vi "Dresden R2R Sputter 03.02.2018 IY24.vi"() -> ()   [LabVIEW 2009] (continued)
                n2407 = local read "RF 1 On"() -> (w4609:bool)
                n2408 = local read "Ch2_Tp_bv_on"() -> (w4633:bool)
                n2409 = local read "Ch2_pressure"() -> (w4594:dbl)
                n2410 = local read "Ch2_Mp_di"() -> (w4632:bool)
                n2411 = Less?(x=w4578, y=0.9) -> (x < y?=w4581:bool)
                n2412 = Less?(x=w4579, y=0.9) -> (x < y?=w4582:bool)
                n2413 = Less?(x=w4575, y=0.9) -> (x < y?=w4572:bool)
                n2414 = Less?(x=w4574, y=0.9) -> (x < y?=w4571:bool)
                n2415 = case shown="True" w4595 {
                  frame #0 {
                    n2416 = local read "Ch2_Pl_atm_di"() -> (w4649:bool)
                    n2417 = case shown="False" w4649 {
                      frame #0 {
                        n2418 = local write "Ch2_Tp_bv_open_safety"(TRUE ("Tp_bv_open_ch1_safety")) -> ()
                      }
                      frame #1 {
                        n2419 = local write "Ch2_Tp_bv_open_safety"(FALSE ("Tp_bv_open_ch1_safety")) -> ()
                      }
                    }
                  }
                  frame #1 {
                    n2420 = local read "Ch2_Pl_atm_di"() -> (w4652:bool)
                    n2421 = case shown="True" w4652 {
                      frame #0 {
                        n2422 = local write "Ch2_Tp_bv_open_safety"(FALSE ("Tp_bv_open_ch1_safety")) -> ()
                      }
                      frame #1 {
                        n2423 = local write "Ch2_Tp_bv_open_safety"(TRUE ("Tp_bv_open_ch1_safety")) -> ()
                      }
                    }
                  }
                }
                n2424 = Less?(x=w4563, y=0.9) -> (x < y?=w4560:bool)
                n2425 = Less?(x=w4562, y=0.9) -> (x < y?=w4559:bool)
                n2426 = Less?(x=w4625, y=0.01) -> (x < y?=w4622:bool)
                n2427 = local read "Ch2_Ds_di"() -> (w4587:bool)
                n2428 = Not(x=w4634) -> (.not. x?=w4635:bool)
                n2429 = Less?(x=w4598, y=0.1) -> (x < y?=w4602:bool)
                n2430 = Less?(x=w4554, y=0.08) -> (x < y?=w4597:bool)
                n2431 = Not(x=w4638) -> (.not. x?=w4637:bool)
                n2432 = Less?(x=w4556, y=0.08) -> (x < y?=w4619:bool)
                n2433 = Not(x=w4623) -> (.not. x?=w4613:bool)
                n2434 = Not And(1:w4601, 2:w4600) -> (0:w4603:bool)
                n2435 = Not(x=w4611) -> (.not. x?=w4610:bool)
                n2436 = Not(x=w4609) -> (.not. x?=w4608:bool)
                n2437 = Not(x=w4647) -> (.not. x?=w4643:bool)
                n2438 = Not(x=w4646) -> (.not. x?=w4644:bool)
                n2439 = Not(x=w4648) -> (.not. x?=w4645:bool)
                n2440 = Less Or Equal?(x=w4626, y=9e-05) -> (x <= y?=w4617:bool)
                n2441 = And(x=w4557, y=w4558) -> (x .and. y?=w4565:bool)
                n2442 = Not Or(1:w4628, 2:w4629) -> (0:w4630:bool)
                n2443 = Less?(x=w4555, y=0.08) -> (x < y?=w4606:bool)
                n2444 = And(x=w4581, y=w4582) -> (x .and. y?=w4584:bool)
                n2445 = Compound Arithmetic op=OR(w4641, w4640) -> (w4639:bool)
                n2446 = And(x=w4572, y=w4571) -> (x .and. y?=w4569:bool)
                n2447 = Less?(x=w4594, y=1.0) -> (x < y?=w4592:bool)
                n2448 = Not(x=w4591) -> (.not. x?=w4590:bool)
                n2449 = Compound Arithmetic op=AND(w4622, w4621, w4619) -> (w4618:bool)
                n2450 = And(x=w4560, y=w4559) -> (x .and. y?=w4566:bool)
                n2451 = And(x=w4602, y=w4603) -> (x .and. y?=w4604:bool)
                n2452 = local write "Ch2_Tp_bv_close_safety"(w4636) -> ()
                n2453 = Compound Arithmetic op=AND(w4645, w4644, w4643, w4607) -> (w4642:bool)
                n2454 = Not(x=w4639) -> (.not. x?=w4588:bool)
                n2455 = Compound Arithmetic op=AND(w4613, w4610, w4608) -> (w4612:bool)
                n2456 = Compound Arithmetic op=OR(w4633, w4632) -> (w4631:bool)
                n2457 = Or(x=w4583, y=w4584) -> (x .or. y?=w4585:bool)
                n2458 = Compound Arithmetic op=AND(w4617, w4616, w4615) -> (→"started_up_ch2":bool)
                n2459 = Or(x=w4570, y=w4569) -> (x .or. y?=w4568:bool)
                n2460 = Or(x=w4565, y=w4566) -> (x .or. y?=w4567:bool)
                n2461 = local write "Ch2_Cc_open_safety"(w4618) -> ()
                n2462 = local write "Ch2_Pl_vbv_open_safety"(w4630) -> ()
                n2463 = Compound Arithmetic op=AND(w4592, w4590) -> (w4589:bool)
                n2464 = local write "Ch2_sov_Ar_open_safety"(w4604) -> ()
                n2465 = local write "Ch2_WFC_close_safety"(w4612) -> ()
                n2466 = local write "Ch2_Ch_vbv_open_safety"(w4642) -> ()
                n2467 = local write "Ch2_sov_Ar_close_safety"(w4606) -> ()
                n2468 = local write "Ch2_Bg_bv_close_safety"(w4597) -> ()
                n2469 = local write "Ch2_Mp_stop_safety"(w4635) -> ()
                n2470 = And(x=w4588, y=w4587) -> (x .and. y?=w4586:bool)
                n2471 = local write "Ch2_Trns_gv_bp2_open_safety"(w4585) -> ()
                n2472 = local write "Ch2_Mp_stop_safety"(w4637) -> ()
                n2473 = local write "Ch2_Trns_gv_bp_open_safety"(w4568) -> ()
                n2474 = local write "Ch2_Bg_bv_open_safety"(w4589) -> ()
                n2475 = local write "Ch2_Tp_start_safety"(w4631) -> ()
                n2476 = local write "Ch2_Mp_start_safety"(w4586) -> ()
                n2477 = local write "Gv_open_ch2_3safety"(w4567) -> ()
              }
              frame #1 {
                w4655 = TRUE
                "Ch2_Bg_bv_open_safety" <- w4655
                "Ch2_Bg_bv_close_safety" <- w4655
                "Ch2_Tp_bv_open_safety" <- w4655
                "Ch2_Tp_bv_close_safety" <- w4655
                "Ch2_Ch_vbv_open_safety" <- w4655
                "Ch2_Ch_vbv_close_safety" <- w4655
                "Ch2_Bp_bv_open_R_safety" <- w4655
                "Ch2_Bp_bv_close_R_safety" <- w4655
                "Ch2_Bp_bv_open_L_safety" <- w4655
                "Ch2_Bp_bv_close_L_safety" <- w4655
                "Ch2_Trns_gv_bp2_open_safety" <- w4655
                "Ch2_Trns_gv_bp2_close_safety" <- w4655
                "Ch2_Trns_gv_bp_open_safety" <- w4655
                "Ch2_Trns_gv_bp_close_safety" <- w4655
                "Ch2_Cc_open_safety" <- w4655
                "Ch2_Cc_close_safety" <- w4655
                "Ch2_sov_Ar_open_safety" <- w4655
                "Ch2_sov_Ar_close_safety" <- w4655
                "Ch2_Mp_start_safety" <- w4655
                "Ch2_Mp_stop_safety" <- w4655
                "Ch2_Pl_vbv_open_safety" <- w4655
                "Ch2_Tp_start_safety" <- w4655
                "Ch2_Tp_stop_safety" <- w4655
                "Ch2_WFC_close_safety" <- w4655
                "Gv_close_ch2_3safety" <- w4655
                "Gv_open_ch2_3safety" <- w4655
              }
            }
            n2478 = case shown="False" "Security_cancel_ch4" {
              frame #0 {
                n2479 = local read "Ch4_Ch_atm_on"() -> (w4490:bool)
                n2480 = local read "Ar_sccm_act 4"() -> (w4485:dbl)
                n2481 = local read "Ch4pressure"() -> (w4538:dbl)
                n2482 = local read "Ar_sccm_act 4"() -> (w4483:dbl)
                n2483 = local read "Ch4pressure"() -> (w4539:dbl)
                n2484 = local read "Ch4_Tp_bv_on"() -> (w4528:bool)
                n2485 = local read "Ch4_Bg_bv_on"() -> (w4530:bool)
                n2486 = local read "Ch4_Ch_vbv_on"() -> (w4487:bool)
                n2487 = local read "TP4_working"() -> (w4523:bool)
                n2488 = local read "Ar_sccm_act 4"() -> (w4484:dbl)
                n2489 = local read "Dcps_is_on"() -> (w4513:bool)
                n2490 = local read "Ch4_Ch_cc_on"() -> (w4529:bool)
                n2491 = local read "Ch4_Tp_bv_on"() -> (w4525:bool)
                n2492 = local read "Ch4_Ch_vbv_on"() -> (w4499:bool)
                n2493 = local read "Tp4_stopped"() -> (w4507:bool)
                n2494 = local read "Ch4_Pc_bv_on"() -> (w4515:bool)
                n2495 = local read "Ch4_Ch_atm_on"() -> (w4498:bool)
                n2496 = local read "TP4_working"() -> (w4521:bool)
                n2497 = local read "Ch4_Pl_vbv_on"() -> (w4541:bool)
                n2498 = local read "RF 1 On"() -> (w4512:bool)
                n2499 = local read "Ch4_Ch_vbv_on"() -> (w4546:bool)
                n2500 = local read "Ch4_Tp_bv_on"() -> (w4544:bool)
                n2501 = local read "Ch4pressure"() -> (w4496:dbl)
                n2502 = local read "TP4_working"() -> (w4516:bool)
                n2503 = local read "Ch4_Mp_di"() -> (w4526:bool)
                n2504 = local read "Ch4pressure"() -> (w4505:dbl)
                n2505 = local read "Ch4_Tp_bv_on"() -> (w4534:bool)
                n2506 = local read "Tp4_stopped"() -> (w4542:bool)
                n2507 = local read "Ch4_Mp_di"() -> (w4535:bool)
                n2508 = case shown="True" w4490 {
                  frame #0 {
                    n2509 = local read "Ch4_Pl_atm_di"() -> (w4547:bool)
                    n2510 = case shown="False" w4547 {
                      frame #0 {
                        n2511 = local write "Ch4_Tp_bv_open_safety"(TRUE ("Tp_bv_open_ch1_safety")) -> ()
                      }
                      frame #1 {
                        n2512 = local write "Ch4_Tp_bv_open_safety"(FALSE ("Tp_bv_open_ch1_safety")) -> ()
                      }
                    }
                  }
                  frame #1 {
                    n2513 = local read "Ch4_Pl_atm_di"() -> (w4550:bool)
                    n2514 = case shown="False" w4550 {
                      frame #0 {
                        n2515 = local write "Ch4_Tp_bv_open_safety"(FALSE ("Tp_bv_open_ch1_safety")) -> ()
                      }
                      frame #1 {
                        n2516 = local write "Ch4_Tp_bv_open_safety"(TRUE ("Tp_bv_open_ch1_safety")) -> ()
                      }
                    }
                  }
                }
                n2517 = Less?(x=w4539, y=0.01) -> (x < y?=w4522:bool)
                n2518 = Less Or Equal?(x=w4538, y=9e-05) -> (x <= y?=w4517:bool)
                n2519 = Not(x=w4512) -> (.not. x?=w4509:bool)
                n2520 = Not(x=w4513) -> (.not. x?=w4510:bool)
                n2521 = Not(x=w4523) -> (.not. x?=w4511:bool)
                n2522 = Less?(x=w4483, y=0.08) -> (x < y?=w4503:bool)
                n2523 = local read "Ch4_Ds_di"() -> (w4492:bool)
                n2524 = Not(x=w4529) -> (.not. x?=w4524:bool)
                n2525 = Less?(x=w4485, y=0.08) -> (x < y?=w4519:bool)
                n2526 = Not(x=w4530) -> (.not. x?=w4532:bool)
                n2527 = Not(x=w4528) -> (.not. x?=w4531:bool)
                n2528 = Less?(x=w4496, y=0.1) -> (x < y?=w4500:bool)
                n2529 = Less?(x=w4484, y=0.08) -> (x < y?=w4495:bool)
                n2530 = Not And(1:w4499, 2:w4498) -> (0:w4501:bool)
                n2531 = Not(x=w4544) -> (.not. x?=w4543:bool)
                n2532 = Less?(x=w4505, y=1.0) -> (x < y?=w4488:bool)
                n2533 = Not Or(1:w4525, 2:w4526) -> (0:w4527:bool)
                n2534 = Not(x=w4487) -> (.not. x?=w4486:bool)
                n2535 = Compound Arithmetic op=OR(w4541, w4546) -> (w4545:bool)
                n2536 = Compound Arithmetic op=AND(w4531, w4532, w4524, w4507) -> (w4533:bool)
                n2537 = Compound Arithmetic op=AND(w4511, w4510, w4509) -> (w4508:bool)
                n2538 = Compound Arithmetic op=AND(w4517, w4516, w4515) -> (→"started_up_ch4":bool)
                n2539 = Compound Arithmetic op=AND(w4522, w4521, w4519) -> (w4518:bool)
                n2540 = Compound Arithmetic op=OR(w4534, w4535) -> (w4536:bool)
                n2541 = And(x=w4500, y=w4501) -> (x .and. y?=w4502:bool)
                n2542 = Not(x=w4545) -> (.not. x?=w4493:bool)
                n2543 = local write "Ch4_Tp_bv_close_safety"(w4542) -> ()
                n2544 = Compound Arithmetic op=AND(w4488, w4486) -> (w4489:bool)
                n2545 = local write "Ch4_Ch_vbv_open_safety"(w4533) -> ()
                n2546 = local write "Ch4_Pl_vbv_open_safety"(w4527) -> ()
                n2547 = local write "Ch4_Bg_bv_close_safety"(w4503) -> ()
                n2548 = local write "Ch4_WFC_close_safety"(w4508) -> ()
                n2549 = local write "Ch4_sov_Ar_close_safety"(w4495) -> ()
                n2550 = local write "Ch4_sov_Ar_open_safety"(w4502) -> ()
                n2551 = And(x=w4493, y=w4492) -> (x .and. y?=w4491:bool)
                n2552 = local write "Ch4_Bg_bv_open_safety"(w4489) -> ()
                n2553 = local write "Ch4_Mp_stop_safety"(w4543) -> ()
                n2554 = local write "Ch4_Cc_open_safety"(w4518) -> ()
                n2555 = local write "Ch4_Tp_start_safety"(w4536) -> ()
                n2556 = local write "Ch4_Mp_start_safety"(w4491) -> ()
              }
              frame #1 {
                w4553 = TRUE
                "Ch4_Bg_bv_open_safety" <- w4553
                "Ch4_Bg_bv_close_safety" <- w4553
                "Ch4_Tp_bv_open_safety" <- w4553
                "Ch4_Tp_bv_close_safety" <- w4553
                "Ch4_Ch_vbv_open_safety" <- w4553
                "Ch4_Ch_vbv_close_safety" <- w4553
                "Ch4_Bp_bv_open_L_safety" <- w4553
                "Ch4_Bp_bv_close_L_safety" <- w4553
                "Ch4_Trns_gv_bp_open_safety" <- w4553
                "Ch4_Trns_gv_bp_close_safety" <- w4553
                "Ch4_Cc_open_safety" <- w4553
                "Ch4_Cc_close_safety" <- w4553
                "Ch4_Mp_start_safety" <- w4553
                "Ch4_Mp_stop_safety" <- w4553
                "Ch4_Pl_vbv_open_safety" <- w4553
                "Ch4_Tp_start_safety" <- w4553
                "Ch4_Tp_stop_safety" <- w4553
                "Ch4_WFC_close_safety" <- w4553
                "Ch4_sov_Ar_open_safety" <- w4553
                "Ch4_sov_Ar_close_safety" <- w4553
              }
            }
            n2557 = case shown="False" "Security_cancel_ch3" {
              frame #0 {
                n2558 = local read "Ar_sccm_act 2"() -> (w4384:dbl)
                n2559 = local read "Ch3_pressure"() -> (w4475:dbl)
                n2560 = local read "Ch3_Ch_atm_on"() -> (w4423:bool)
                n2561 = local read "Ch3_Ch_vbv_on"() -> (w4457:bool)
                n2562 = local read "Ar_sccm_act 2"() -> (w4385:dbl)
                n2563 = local read "Ch3_Pl_vbv_on"() -> (w4458:bool)
                n2564 = local read "Ch3_Ds_di"() -> (w4421:bool)
                n2565 = local read "Ch3_Tp_bv_on"() -> (w4465:bool)
                n2566 = local read "Ch3_Bg_bv_on"() -> (w4463:bool)
                n2567 = local read "Ch3_Ch_cc_on"() -> (w4464:bool)
                n2568 = local read "Ch4_pressure2"() -> (w4395:dbl)
                n2569 = local read "Ch3_Ch_vbv_on"() -> (w4419:bool)
                n2570 = local read "Ch3_pressure2"() -> (w4394:dbl)
                n2571 = local read "Ch3_pressure2"() -> (w4398:dbl)
                n2572 = local read "Ch3_Tp_bv_on"() -> (w4468:bool)
                n2573 = local read "TP3_working"() -> (w4452:bool)
                n2574 = local read "Ch3_Ch_vbv_on"() -> (w4431:bool)
                n2575 = local read "Ch4_pressure2"() -> (w4399:dbl)
                n2576 = local read "Ch3_Tp_bv_on"() -> (w4424:bool)
                n2577 = local read "Ch3_pressure"() -> (w4472:dbl)
                n2578 = local read "TP3_working"() -> (w4455:bool)
                n2579 = local read "TP3_working"() -> (w4444:bool)
                n2580 = local read "TP3_working"() -> (w4443:bool)
                n2581 = local read "Tp3_stopped"() -> (w4445:bool)
                n2582 = local read "Ch3_Ch_atm_on"() -> (w4432:bool)
                n2583 = local read "Ch3_pressure2"() -> (w4409:dbl)
                n2584 = local read "Ch3_pressure"() -> (w4434:dbl)
                n2585 = local read "Ch4_pressure2"() -> (w4410:dbl)
                n2586 = local read "Ch3_Ch_atm_on"() -> (w4390:bool)
                n2587 = local read "Ch4_Ch_atm_on"() -> (w4414:bool)
                n2588 = local read "Ch3_Ch_atm_on"() -> (w4415:bool)
                n2589 = local read "Ch3_Tp_bv_on"() -> (w4471:bool)
                n2590 = local read "Ch3_Ch_atm_on"() -> (w4403:bool)
                n2591 = local read "Ch3_Pc_bv_on"() -> (w4447:bool)
                n2592 = local read "Ch3_Mp_di"() -> (w4467:bool)
                n2593 = local read "Ch3_pressure"() -> (w4437:dbl)
                n2594 = local read "Tp3_stopped"() -> (w4454:bool)
                n2595 = local read "TP3_working"() -> (w4448:bool)
                n2596 = local read "Ar_sccm_act 2"() -> (w4383:dbl)
                n2597 = local read "Ch3_Mp_di"() -> (w4470:bool)
                n2598 = Less?(x=w4475, y=0.01) -> (x < y?=w4453:bool)
                n2599 = Not(x=w4464) -> (.not. x?=w4460:bool)
                n2600 = Not(x=w4463) -> (.not. x?=w4461:bool)
                n2601 = Not(x=w4465) -> (.not. x?=w4462:bool)
                n2602 = Less?(x=w4385, y=0.08) -> (x < y?=w4451:bool)
                n2603 = Not(x=w4443) -> (.not. x?=w4440:bool)
                n2604 = Not(x=w4455) -> (.not. x?=w4442:bool)
                n2605 = Not(x=w4444) -> (.not. x?=w4441:bool)
                n2606 = Less?(x=w4395, y=0.9) -> (x < y?=w4392:bool)
                n2607 = Less?(x=w4394, y=0.9) -> (x < y?=w4391:bool)
                n2608 = Less?(x=w4398, y=0.9) -> (x < y?=w4401:bool)
                n2609 = Less?(x=w4399, y=0.9) -> (x < y?=w4402:bool)
                n2610 = Not(x=w4424) -> (.not. x?=w4425:bool)
                n2611 = Compound Arithmetic op=OR(w4458, w4457) -> (w4456:bool)
                n2612 = Less?(x=w4409, y=0.9) -> (x < y?=w4412:bool)
                n2613 = case shown="False" w4423 {
                  frame #0 {
                    n2614 = local read "Ch3_Pl_atm_di"() -> (w4476:bool)
                    n2615 = case shown="False" w4476 {
                      frame #0 {
                        n2616 = local write "Ch3_Tp_bv_open_safety"(TRUE ("Tp_bv_open_ch1_safety")) -> ()
                      }
                      frame #1 {
                        n2617 = local write "Ch3_Tp_bv_open_safety"(FALSE ("Tp_bv_open_ch1_safety")) -> ()
                      }
                    }
                  }
                  frame #1 {
                    n2618 = local read "Ch3_Pl_atm_di"() -> (w4479:bool)
                    n2619 = case shown="True" w4479 {
                      frame #0 {
                        n2620 = local write "Ch3_Tp_bv_open_safety"(FALSE ("Tp_bv_open_ch1_safety")) -> ()
                      }
                      frame #1 {
                        n2621 = local write "Ch3_Tp_bv_open_safety"(TRUE ("Tp_bv_open_ch1_safety")) -> ()
                      }
                    }
                  }
                }
                n2622 = Less?(x=w4434, y=0.1) -> (x < y?=w4430:bool)
                n2623 = Less?(x=w4384, y=0.08) -> (x < y?=w4435:bool)
                n2624 = Less?(x=w4410, y=0.9) -> (x < y?=w4413:bool)
                n2625 = Not And(1:w4431, 2:w4432) -> (0:w4429:bool)
                n2626 = Not Or(1:w4468, 2:w4467) -> (0:w4466:bool)
                n2627 = Less?(x=w4437, y=0.1) -> (x < y?=w4418:bool)
                n2628 = Not(x=w4419) -> (.not. x?=w4417:bool)
                n2629 = Less Or Equal?(x=w4472, y=9e-05) -> (x <= y?=w4449:bool)
                n2630 = Compound Arithmetic op=AND(w4462, w4461, w4460, w4445) -> (w4459:bool)
                n2631 = Less?(x=w4383, y=0.08) -> (x < y?=w4426:bool)
                n2632 = Not(x=w4456) -> (.not. x?=w4422:bool)
                n2633 = Compound Arithmetic op=OR(w4471, w4470) -> (w4469:bool)
                n2634 = Compound Arithmetic op=AND(w4442, w4441, w4440) -> (w4439:bool)
                n2635 = Compound Arithmetic op=AND(w4453, w4452, w4451) -> (w4450:bool)
                n2636 = And(x=w4430, y=w4429) -> (x .and. y?=w4428:bool)
                n2637 = And(x=w4415, y=w4414) -> (x .and. y?=w4407:bool)
                n2638 = local write "Ch3_Tp_bv_close_safety"(w4454) -> ()
                n2639 = And(x=w4392, y=w4391) -> (x .and. y?=w4389:bool)
                n2640 = And(x=w4422, y=w4421) -> (x .and. y?=w4420:bool)
                n2641 = And(x=w4401, y=w4402) -> (x .and. y?=w4404:bool)
                n2642 = local write "Ch3_Ch_vbv_open_safety"(w4459) -> ()
                n2643 = Compound Arithmetic op=AND(w4449, w4448, w4447) -> (→"started_up_ch3":bool)
                n2644 = And(x=w4412, y=w4413) -> (x .and. y?=w4387:bool)
                n2645 = local write "Ch3_Pl_vbv_open_safety"(w4466) -> ()
                n2646 = local write "Ch3_WFC_close_safety"(w4439) -> ()
                n2647 = local write "Ch3_sov_Ar_open_safety"(w4428) -> ()
                n2648 = Compound Arithmetic op=AND(w4418, w4417) -> (w4416:bool)
                n2649 = Or(x=w4390, y=w4389) -> (x .or. y?=w4388:bool)
                n2650 = Or(x=w4403, y=w4404) -> (x .or. y?=w4405:bool)
                n2651 = local write "Ch3_Mp_stop_safety"(w4425) -> ()
                n2652 = local write "Ch3_Bg_bv_close_safety"(w4435) -> ()
                n2653 = local write "Ch3_sov_Ar_close_safety"(w4426) -> ()
                n2654 = local write "Ch3_Cc_open_safety"(w4450) -> ()
                n2655 = Or(x=w4407, y=w4387) -> (x .or. y?=w4406:bool)
                n2656 = local write "Ch3_Tp_start_safety"(w4469) -> ()
                n2657 = local write "Ch3_Mp_start_safety"(w4420) -> ()
                n2658 = local write "Ch3_Trns_gv_bp2_open_safety"(w4388) -> ()
                n2659 = local write "Ch3_Trns_gv_bp_open_safety"(w4405) -> ()
                n2660 = local write "Ch3_Bg_bv_start_safety"(w4416) -> ()
                n2661 = local write "Gv_open_ch3_4safety"(w4406) -> ()
              }
              frame #1 {
                w4482 = TRUE
                "Ch3_Bg_bv_start_safety" <- w4482
                "Ch3_Bg_bv_close_safety" <- w4482
                "Ch3_Tp_bv_open_safety" <- w4482
                "Ch3_Tp_bv_close_safety" <- w4482
                "Ch3_Ch_vbv_open_safety" <- w4482
                "Ch3_Ch_vbv_close_safety" <- w4482
                "Ch3_Bp_bv_open_R_safety" <- w4482
                "Ch3_Bp_bv_close_R_safety" <- w4482
                "Ch3_Bp_bv_close_L_safety" <- w4482
                "Ch3_Bp_bv_open_L_safety" <- w4482
                "Ch3_Trns_gv_bp2_close_safety" <- w4482
                "Ch3_Trns_gv_bp2_open_safety" <- w4482
                "Ch3_Trns_gv_bp_open_safety" <- w4482
                "Ch3_Trns_gv_bp_close_safety" <- w4482
                "Ch3_Cc_open_safety" <- w4482
                "Ch3_Cc_close_safety" <- w4482
                "Ch3_sov_Ar_open_safety" <- w4482
                "Ch3_sov_Ar_close_safety" <- w4482
                "Ch3_Mp_start_safety" <- w4482
                "Ch3_Mp_stop_safety" <- w4482
                "Ch3_Pl_vbv_open_safety" <- w4482
                "Ch3_Tp_start_safety" <- w4482
                "Ch3_Tp_stop_safety" <- w4482
                "Ch3_WFC_close_safety" <- w4482
                "Gv_open_ch3_4safety" <- w4482
                "Gv_close_ch3_4safety" <- w4482
              }
            }
          }
        }
        n2662 = stacked-sequence {
          frame #0 {
            # "GAS FLOW CONTROL"
            n2663 = Or(x="Ar_set_zero_ch1", y="Ar_auto_set_zero_ch1") -> (x .or. y?=w4321:bool)
            n2664 = Or(x="Ar_set_zero_ch2", y="Ar_auto_set_zero_ch2") -> (x .or. y?=w4311:bool)
            n2665 = case shown="True" "Mfc_Ar _set 2" {
              frame #0 {
              }
              frame #1 {
                n2666 = stacked-sequence {
                  frame #0 {
                    n2667 = local write "Ar_sccm1_2"(u16 0 ("Ar_sccm 2")) -> ()
                  }
                  frame #1 {
                    n2668 = Wait (ms)(milliseconds to wait=u32 200) -> ()  [unwired: 1 out]
                  }
                  frame #2 {
                    n2669 = local write "Mfc_Ar _1_2_set"(TRUE ("Ar_set_ch1")) -> ()
                  }
                  frame #3 {
                    n2670 = Wait (ms)(milliseconds to wait=u32 1000) -> ()  [unwired: 1 out]
                  }
                  frame #4 {
                    n2671 = local write "Mfc_Ar _1_2_set"(FALSE ("Ar_set_ch1")) -> ()
                  }
                  frame #5 {
                    n2672 = Wait (ms)(milliseconds to wait=u32 200) -> ()  [unwired: 1 out]
                  }
                  frame #6 {
                    n2673 = local write "Ar_sccm1_2"("Ar_sccm 2") -> ()
                  }
                  frame #7 {
                    n2674 = Wait (ms)(milliseconds to wait=u32 200) -> ()  [unwired: 1 out]
                  }
                  frame #8 {
                    n2675 = local write "Mfc_Ar _1_2_set"(TRUE ("Ar_set_ch1")) -> ()
                  }
                  frame #9 {
                    n2676 = Wait (ms)(milliseconds to wait=u32 1000) -> ()  [unwired: 1 out]
                  }
                  frame #10 {
                    n2677 = local write "Mfc_Ar _set 2"(FALSE ("Mfc_Ar _set 2")) -> ()
                  }
                }
              }
            }
            n2678 = case shown="True" w4311 {
              frame #0 {
              }
              frame #1 {
                n2679 = flat-sequence {
                  frame #0 {
                    n2680 = local write "Ar_sccm1_2"(u16 0 ("Ar_sccm 2")) -> ()
                  }
                  frame #1 {
                    n2681 = Wait (ms)(milliseconds to wait=u32 200) -> ()  [unwired: 1 out]
                  }
                  frame #2 {
                    n2682 = local write "Ar_auto_set_zero_ch2"(FALSE ("Ar_auto_set_zero_ch2")) -> ()
                    n2683 = local write "Mfc_Ar _1_2_set"(TRUE ("Ar_set_ch1")) -> ()
                  }
                }
              }
            }
            n2684 = case shown="True" w4321 {
              frame #0 {
              }
              frame #1 {
                n2685 = flat-sequence {
                  frame #0 {
                    n2686 = local write "Ar_sccm1_2"(u16 0 ("Ar_sccm 2")) -> ()
                  }
                  frame #1 {
                    n2687 = Wait (ms)(milliseconds to wait=u32 200) -> ()  [unwired: 1 out]
                  }
                  frame #2 {
                    n2688 = local write "Ar_auto_set_zero_ch1"(FALSE ("Ar_auto_set_zero_ch1")) -> ()
                    n2689 = local write "Mfc_Ar _1_2_set"(TRUE ("Ar_set_ch1")) -> ()
                  }
                }
              }
            }
            n2690 = case shown="True" "Mfc2_Ar _set4" {
              frame #0 {
              }
              frame #1 {
                n2691 = stacked-sequence {
                  frame #0 {
                    n2692 = local write "Ar_sccm3_4"(u16 0 ("Ar_sccm3_4")) -> ()
                  }
                  frame #1 {
                    n2693 = Wait (ms)(milliseconds to wait=u32 200) -> ()  [unwired: 1 out]
                  }
                  frame #2 {
                    n2694 = local write "Mfc2_Ar _3_4_set"(TRUE ("Mfc2_Ar _set")) -> ()
                  }
                  frame #3 {
                    n2695 = Wait (ms)(milliseconds to wait=u32 1000) -> ()  [unwired: 1 out]
                  }
                  frame #4 {
                    n2696 = local write "Ar_sccm3_4"("Ar_sccm4") -> ()
                  }
                  frame #5 {
                    n2697 = Wait (ms)(milliseconds to wait=u32 200) -> ()  [unwired: 1 out]
                  }
                  frame #6 {
                    n2698 = local write "Mfc2_Ar _3_4_set"(TRUE ("Mfc2_Ar _set")) -> ()
                  }
                  frame #7 {
                    n2699 = Wait (ms)(milliseconds to wait=u32 1000) -> ()  [unwired: 1 out]
                  }
                  frame #8 {
                    n2700 = local write "Mfc2_Ar _set4"(FALSE ("Mfc2_Ar _set4")) -> ()
                  }
                }
              }
            }
            n2701 = case shown="True" "Mfc_Ar _set" {
              frame #0 {
              }
              frame #1 {
                n2702 = stacked-sequence {
                  frame #0 {
                    n2703 = local write "Ar_sccm1_2"(u16 0 ("Ar_sccm 2")) -> ()
                  }
                  frame #1 {
                    n2704 = Wait (ms)(milliseconds to wait=u32 200) -> ()  [unwired: 1 out]
                  }
                  frame #2 {
                    n2705 = local write "Mfc_Ar _1_2_set"(TRUE ("Ar_set_ch1")) -> ()
                  }
                  frame #3 {
                    n2706 = Wait (ms)(milliseconds to wait=u32 1000) -> ()  [unwired: 1 out]
                  }
                  frame #4 {
                    n2707 = local write "Mfc_Ar _1_2_set"(FALSE ("Ar_set_ch1")) -> ()
                  }
                  frame #5 {
                    n2708 = Wait (ms)(milliseconds to wait=u32 200) -> ()  [unwired: 1 out]
                  }
                  frame #6 {
                    n2709 = local write "Ar_sccm1_2"("Ar_sccm") -> ()
                  }
                  frame #7 {
                    n2710 = Wait (ms)(milliseconds to wait=u32 200) -> ()  [unwired: 1 out]
                  }
                  frame #8 {
                    n2711 = local write "Mfc_Ar _1_2_set"(TRUE ("Ar_set_ch1")) -> ()
                  }
                  frame #9 {
                    n2712 = Wait (ms)(milliseconds to wait=u32 1000) -> ()  [unwired: 1 out]
                  }
                  frame #10 {
                    n2713 = local write "Mfc_Ar _set"(FALSE ("Mfc_Ar _set")) -> ()
                  }
                }
              }
            }
            n2714 = case shown="True" "Mfc2_Ar _set3" {
              frame #0 {
              }
              frame #1 {
                n2715 = stacked-sequence {
                  frame #0 {
                    n2716 = local write "Ar_sccm3_4"(u16 0 ("Ar_sccm3_4")) -> ()
                  }
                  frame #1 {
                    n2717 = Wait (ms)(milliseconds to wait=u32 200) -> ()  [unwired: 1 out]
                  }
                  frame #2 {
                    n2718 = local write "Mfc2_Ar _3_4_set"(TRUE ("Mfc2_Ar _set")) -> ()
                  }
                  frame #3 {
                    n2719 = Wait (ms)(milliseconds to wait=u32 1000) -> ()  [unwired: 1 out]
                  }
                  frame #4 {
                    n2720 = local write "Ar_sccm3_4"("Ar_sccm3") -> ()
                  }
                  frame #5 {
                    n2721 = Wait (ms)(milliseconds to wait=u32 200) -> ()  [unwired: 1 out]
                  }
                  frame #6 {
                    n2722 = local write "Mfc2_Ar _3_4_set"(TRUE ("Mfc2_Ar _set")) -> ()
                  }
                  frame #7 {
                    n2723 = Wait (ms)(milliseconds to wait=u32 1000) -> ()  [unwired: 1 out]
                  }
                  frame #8 {
                    n2724 = local write "Mfc2_Ar _set3"(FALSE ("Mfc2_Ar _set3")) -> ()
                  }
                }
              }
            }
            n2725 = Or(x="Ar_set_zero_ch4", y="Ar_auto_set_zero_ch4") -> (x .or. y?=w4313:bool)
            n2726 = Or(x="Ar_set_zero_ch3", y="Ar_auto_set_zero_ch3") -> (x .or. y?=w4316:bool)
            n2727 = case shown="True" w4313 {
              frame #0 {
              }
              frame #1 {
                n2728 = flat-sequence {
                  frame #0 {
                    n2729 = local write "Ar_sccm3_4"(u16 0 ("Ar_sccm2 2")) -> ()
                  }
                  frame #1 {
                    n2730 = Wait (ms)(milliseconds to wait=u32 200) -> ()  [unwired: 1 out]
                  }
                  frame #2 {
                    n2731 = local write "Mfc2_Ar _3_4_set"(TRUE ("Mfc2_Ar _set")) -> ()
                    n2732 = local write "Ar_auto_set_zero_ch4"(FALSE ("Ar_auto_set_zero_ch4")) -> ()
                  }
                }
              }
            }
            n2733 = case shown="True" w4316 {
              frame #0 {
              }
              frame #1 {
                n2734 = flat-sequence {
                  frame #0 {
                    n2735 = local write "Ar_sccm3_4"(u16 0 ("Ar_sccm2 2")) -> ()
                  }
                  frame #1 {
                    n2736 = Wait (ms)(milliseconds to wait=u32 200) -> ()  [unwired: 1 out]
                  }
                  frame #2 {
                    n2737 = local write "Ar_auto_set_zero_ch3"(FALSE ("Ar_auto_set_zero_ch3")) -> ()
                    n2738 = local write "Mfc2_Ar _3_4_set"(TRUE ("Mfc2_Ar _set")) -> ()
                  }
                }
              }
            }
          }
        }
        n2739 = stacked-sequence {
          frame #0 {
            # "Process Flow"
            n2740 = case shown="True" "Ppsok" {
              frame #0 {
              }
              frame #1 {
                n2741 = stacked-sequence {
                  frame #0 {
                    n2742 = local read "Pps_code_entry"() -> (w5512:string)
                    n2743 = Equal?(x=w5512, y="PF227= ") -> (x = y?=w5510:bool)
                    n2744 = Read from Text File(file (use dialog)="Process_flow_messages") -> (text=w5520:string)  [unwired: 3 in, 3 out]
                    n2745 = Match Pattern(string=w5520, regular expression="Pps_code_entry") -> (after substring=w5521:string)  [unwired: 1 in, 3 out]
                    n2746 = case shown="False" w5510 {
                      tunnel: [w5522 "                "] -> w5509
                      frame #0 {
                        n2747 = Get Date/Time String() -> (date string=w5525:string, time string=w5523:string)  [unwired: 3 in]
                        n2748 = Concatenate Strings(w5525, " / " ("string"), w5523) -> (w5522:string)
                      }
                      frame #1 {
                      }
                    }
                    n2749 = Match Pattern(string=w5521, regular expression="***") -> (before substring=w5516:string)  [unwired: 1 in, 3 out]
                    n2750 = Concatenate Strings(w5509, w5516) -> (w5514:string)
                    n2751 = String Length(string=w5516) -> (length=w5517:i32)
                    n2752 = Not Equal To 0?(x=w5517) -> (x != 0?=w5515:bool)
                    n2753 = case shown="True" w5515 {
                      tunnel: w5514 -> [_ w5532]
                      frame #0 {
                      }
                      frame #1 {
                        n2754 = property on="Process_flow" class="Str"() -> ("Text.Scroll Position"=w5529:u32)  [unwired: 2 in, 2 out]
                        n2755 = local read "Process_flow"() -> (w5530:string)
                        n2756 = Concatenate Strings(w5530, "\r", w5532) -> (w5527:string)
                        n2757 = Add(x=w5529, y=u32 10) -> (x+y=w5528:u32)
                        n2758 = local write "Process_flow"(w5527) -> ()
                        n2759 = property on="Process_flow" class="Str"("Text.Scroll Position"=w5528) -> ()  [unwired: 2 in, 2 out]
                      }
                    }
                  }
                  frame #1 {
                    n2760 = Wait (ms)(milliseconds to wait=u32 100) -> ()  [unwired: 1 out]
                  }
                  frame #2 {
                    n2761 = local write "Ppsok"(FALSE ("PPSOK")) -> ()
                  }
                }
              }
            }
          }
        }
        n2762 = stacked-sequence {
          frame #0 {
            # "INSTANT MESSAGES"
            n2763 = local read "Ch3_Ch_vbv_on"() -> (w4843:bool)
            n2764 = local read "Ch3_Bp_bv_on_L"() -> (w4908:bool)
            n2765 = local read "Ch3_Pl_atm_on"() -> (w4854:bool)
            n2766 = local read "Ch4_Ch_vbv_on"() -> (w4824:bool)
            n2767 = local read "Ch2_Ch_vbv_on"() -> (w4984:bool)
            n2768 = local read "Ch2_Bp_bv_on_L"() -> (w4919:bool)
            n2769 = local read "Ch4_Pl_atm_on"() -> (w4813:bool)
            n2770 = local read "Ch2_Pl_atm_on"() -> (w4973:bool)
            n2771 = local read "Ch1_Ch_vbv_on"() -> (w5013:bool)
            n2772 = local read "Ch1_Pl_atm_on"() -> (w5024:bool)
            n2773 = local read "Ch3_Pl_pg_on"() -> (w4873:bool)
            n2774 = local read "Ch4_Pl_pg_on"() -> (w4794:bool)
            n2775 = local read "Ch2_Pl_pg_on"() -> (w4954:bool)
            n2776 = local read "Ch3_Pl_vbv_on"() -> (w4894:bool)
            n2777 = local read "Ch4_Pl_vbv_on"() -> (w4773:bool)
            n2778 = local read "Ch2_Pl_vbv_on"() -> (w4933:bool)
            n2779 = local read "Ch1_Pl_pg_on"() -> (w5043:bool)
            n2780 = local read "Ch1_Pl_vbv_on"() -> (w5064:bool)
            n2781 = local read "Ch3_Mp_on"() -> (w4899:bool)
            n2782 = local read "Ch4_Mp_on"() -> (w4768:bool)
            n2783 = local read "Ch2_Mp_on"() -> (w4928:bool)
            n2784 = local read "Ch1_Mp_on"() -> (w5069:bool)
            n2785 = feedback #54() -> (w4855:bool)  [unwired: 1 in]
            n2786 = feedback #55() -> (w4842:bool)  [unwired: 1 in]
            n2787 = feedback #56() -> (w4812:bool)  [unwired: 1 in]
            n2788 = feedback #57() -> (w4972:bool)  [unwired: 1 in]
            n2789 = feedback #58() -> (w4825:bool)  [unwired: 1 in]
            n2790 = feedback #59() -> (w4985:bool)  [unwired: 1 in]
            n2791 = feedback #60() -> (w4872:bool)  [unwired: 1 in]
            n2792 = feedback #61() -> (w4907:bool)  [unwired: 1 in]
            n2793 = feedback #62() -> (w4795:bool)  [unwired: 1 in]
            n2794 = feedback #63() -> (w5025:bool)  [unwired: 1 in]
            n2795 = feedback #64() -> (w4955:bool)  [unwired: 1 in]
            n2796 = feedback #65() -> (w4920:bool)  [unwired: 1 in]
            n2797 = feedback #66() -> (w5012:bool)  [unwired: 1 in]
            n2798 = feedback #67() -> (w4903:bool)  [unwired: 1 in]
            n2799 = feedback #68() -> (w4895:bool)  [unwired: 1 in]
            n2800 = feedback #69() -> (w5042:bool)  [unwired: 1 in]
            n2801 = feedback #70() -> (w4764:bool)  [unwired: 1 in]
            n2802 = feedback #71() -> (w4772:bool)  [unwired: 1 in]
            n2803 = feedback #72() -> (w4924:bool)  [unwired: 1 in]
            n2804 = feedback #73() -> (w4932:bool)  [unwired: 1 in]
            n2805 = feedback #74() -> (w5073:bool)  [unwired: 1 in]
            n2806 = feedback #75() -> (w5065:bool)  [unwired: 1 in]
            n2807 = Boolean To (0,1)(Boolean=w4854) -> (0, 1=w4856:i16)
            n2808 = Boolean To (0,1)(Boolean=w4855) -> (0, 1=w4857:i16)
            n2809 = Boolean To (0,1)(Boolean=w4843) -> (0, 1=w4841:i16)
            n2810 = Boolean To (0,1)(Boolean=w4842) -> (0, 1=w4840:i16)
            n2811 = Boolean To (0,1)(Boolean=w4813) -> (0, 1=w4811:i16)
            n2812 = Boolean To (0,1)(Boolean=w4812) -> (0, 1=w4810:i16)
            n2813 = Boolean To (0,1)(Boolean=w4973) -> (0, 1=w4971:i16)
            n2814 = Boolean To (0,1)(Boolean=w4972) -> (0, 1=w4970:i16)
            n2815 = Boolean To (0,1)(Boolean=w4824) -> (0, 1=w4826:i16)
            n2816 = Boolean To (0,1)(Boolean=w4825) -> (0, 1=w4827:i16)
            n2817 = Boolean To (0,1)(Boolean=w4984) -> (0, 1=w4986:i16)
            n2818 = Boolean To (0,1)(Boolean=w4985) -> (0, 1=w4987:i16)
            n2819 = Boolean To (0,1)(Boolean=w4873) -> (0, 1=w4871:i16)
            n2820 = Boolean To (0,1)(Boolean=w4872) -> (0, 1=w4870:i16)
            n2821 = Boolean To (0,1)(Boolean=w4908) -> (0, 1=w4906:i16)
            n2822 = Boolean To (0,1)(Boolean=w4907) -> (0, 1=w4905:i16)
            n2823 = Boolean To (0,1)(Boolean=w4794) -> (0, 1=w4796:i16)
            n2824 = Boolean To (0,1)(Boolean=w4795) -> (0, 1=w4797:i16)
            n2825 = Boolean To (0,1)(Boolean=w5024) -> (0, 1=w5026:i16)
            n2826 = Boolean To (0,1)(Boolean=w5025) -> (0, 1=w5027:i16)
            n2827 = Boolean To (0,1)(Boolean=w4954) -> (0, 1=w4956:i16)
            n2828 = Boolean To (0,1)(Boolean=w4955) -> (0, 1=w4957:i16)
            n2829 = Boolean To (0,1)(Boolean=w4919) -> (0, 1=w4921:i16)
            n2830 = Boolean To (0,1)(Boolean=w4920) -> (0, 1=w4922:i16)
            n2831 = Boolean To (0,1)(Boolean=w5013) -> (0, 1=w5011:i16)
            n2832 = Boolean To (0,1)(Boolean=w5012) -> (0, 1=w5010:i16)
            n2833 = Boolean To (0,1)(Boolean=w4899) -> (0, 1=w4902:i16)
            n2834 = Boolean To (0,1)(Boolean=w4903) -> (0, 1=w4901:i16)
            n2835 = Boolean To (0,1)(Boolean=w4894) -> (0, 1=w4896:i16)
            n2836 = Boolean To (0,1)(Boolean=w4895) -> (0, 1=w4897:i16)
            n2837 = Boolean To (0,1)(Boolean=w5043) -> (0, 1=w5041:i16)
            n2838 = Boolean To (0,1)(Boolean=w5042) -> (0, 1=w5040:i16)
            n2839 = Boolean To (0,1)(Boolean=w4768) -> (0, 1=w4765:i16)
            n2840 = Boolean To (0,1)(Boolean=w4764) -> (0, 1=w4766:i16)
            n2841 = Boolean To (0,1)(Boolean=w4773) -> (0, 1=w4771:i16)
            n2842 = Boolean To (0,1)(Boolean=w4772) -> (0, 1=w4770:i16)
            n2843 = Boolean To (0,1)(Boolean=w4928) -> (0, 1=w4925:i16)
            n2844 = Boolean To (0,1)(Boolean=w4924) -> (0, 1=w4926:i16)
            n2845 = Boolean To (0,1)(Boolean=w4933) -> (0, 1=w4931:i16)
            n2846 = Boolean To (0,1)(Boolean=w4932) -> (0, 1=w4930:i16)
            n2847 = Boolean To (0,1)(Boolean=w5069) -> (0, 1=w5072:i16)
            n2848 = Boolean To (0,1)(Boolean=w5073) -> (0, 1=w5071:i16)
            n2849 = Boolean To (0,1)(Boolean=w5064) -> (0, 1=w5066:i16)
            n2850 = Boolean To (0,1)(Boolean=w5065) -> (0, 1=w5067:i16)
            n2851 = Not Equal?(x=w4856, y=w4857) -> (x != y?=w4858:bool)
            n2852 = Not Equal?(x=w4841, y=w4840) -> (x != y?=w4839:bool)
            n2853 = Not Equal?(x=w4811, y=w4810) -> (x != y?=w4809:bool)
            n2854 = Not Equal?(x=w4971, y=w4970) -> (x != y?=w4969:bool)
            n2855 = Not Equal?(x=w4826, y=w4827) -> (x != y?=w4828:bool)
            n2856 = Not Equal?(x=w4986, y=w4987) -> (x != y?=w4988:bool)
            n2857 = Not Equal?(x=w4871, y=w4870) -> (x != y?=w4869:bool)
            n2858 = Not Equal?(x=w4906, y=w4905) -> (x != y?=w4904:bool)
            n2859 = Not Equal?(x=w4796, y=w4797) -> (x != y?=w4798:bool)
            n2860 = Not Equal?(x=w5026, y=w5027) -> (x != y?=w5028:bool)
            n2861 = Not Equal?(x=w4956, y=w4957) -> (x != y?=w4958:bool)
            n2862 = Not Equal?(x=w4921, y=w4922) -> (x != y?=w4923:bool)
            n2863 = Not Equal?(x=w5011, y=w5010) -> (x != y?=w5009:bool)
            n2864 = Not Equal?(x=w4902, y=w4901) -> (x != y?=w4900:bool)
            n2865 = Not Equal?(x=w4896, y=w4897) -> (x != y?=w4898:bool)
            n2866 = Not Equal?(x=w5041, y=w5040) -> (x != y?=w5039:bool)
            n2867 = Not Equal?(x=w4765, y=w4766) -> (x != y?=w4767:bool)
            n2868 = Not Equal?(x=w4771, y=w4770) -> (x != y?=w4769:bool)
            n2869 = Not Equal?(x=w4925, y=w4926) -> (x != y?=w4927:bool)
            n2870 = Not Equal?(x=w4931, y=w4930) -> (x != y?=w4929:bool)
            n2871 = Not Equal?(x=w5072, y=w5071) -> (x != y?=w5070:bool)
            n2872 = Not Equal?(x=w5066, y=w5067) -> (x != y?=w5068:bool)
            n2873 = case shown="True" w4858 {
              tunnel: w4854 -> [_ w5214]
              frame #0 {
              }
              frame #1 {
                n2874 = case shown="False" w5214 {
                  frame #0 {
                    n2875 = stacked-sequence {
                      frame #0 {
                        n2876 = local write "Pps_code_entry"("PF172=" ("Pps_code_entry")) -> ()
                      }
                      frame #1 {
                        n2877 = Wait (ms)(milliseconds to wait=u32 500) -> ()  [unwired: 1 out]
                      }
                      frame #2 {
                        n2878 = local write "Ppsok"(TRUE ("Ppsok")) -> ()
                      }
                    }
                  }
                  frame #1 {
                    n2879 = stacked-sequence {
                      frame #0 {
                        n2880 = local write "Pps_code_entry"("PF171=" ("Pps_code_entry")) -> ()
                      }
                      frame #1 {
                        n2881 = Wait (ms)(milliseconds to wait=u32 500) -> ()  [unwired: 1 out]
                      }
                      frame #2 {
                        n2882 = local write "Ppsok"(TRUE ("Ppsok")) -> ()
                      }
                    }
                  }
                }
              }
            }
            n2883 = case shown="True" w4839 {
              tunnel: w4843 -> [_ w5193]
              frame #0 {
              }
              frame #1 {
                n2884 = case shown="True" w5193 {
                  frame #0 {